vi "UHR-Fleezers Control (host) - 12.8.vi"() -> ()   [LabVIEW 2012] (continued)
                                }
                                }
                                frame #4 {
                                n2130 = Wait (ms)(milliseconds to wait=u32 500) -> ()  [unwired: 1 out]
                                }
                                frame #5 {
                                n2131 = local read "Mean"() -> (w3230:dbl)
                                n2132 = Greater?(x=w3230, y=11.0) -> (0:w3224:bool)
                                n2133 = Not(x=w3224) -> (.not. x?=w3225:bool)
                                n2134 = And(x=w3225, y="Shift confocal") -> (x .and. y?=w3227:bool)
                                n2135 = And(x=w3224, y="Shift confocal") -> (x .and. y?=w3228:bool)
                                n2136 = case shown="True" w3228 {
                                frame False {
                                }
                                frame True {
                                n2137 = local read "Confocal Y 2 (V)"() -> (w3234:dbl)
                                n2138 = local read "Confocal X 2 (V)"() -> (w3233:dbl)
                                n2139 = property on="AO1" class="Slide (strict)"("Val(Sgnl)"=w3234) -> ()  [unwired: 2 in, 2 out]
                                n2140 = property on="AO2" class="Slide (strict)"("Val(Sgnl)"=w3233) -> ()  [unwired: 2 in, 2 out]
                                }
                                }
                                n2141 = case shown="True" w3227 {
                                frame False {
                                }
                                frame True {
                                n2142 = local read "Confocal Y 1 (V)"() -> (w3232:dbl)
                                n2143 = local read "Confocal X 1 (V)"() -> (w3231:dbl)
                                n2144 = property on="AO1" class="Slide (strict)"("Val(Sgnl)"=w3232) -> ()  [unwired: 2 in, 2 out]
                                n2145 = property on="AO2" class="Slide (strict)"("Val(Sgnl)"=w3231) -> ()  [unwired: 2 in, 2 out]
                                }
                                }
                                }
                                frame #6 {
                                n2146 = Wait (ms)(milliseconds to wait=u32 1500) -> ()  [unwired: 1 out]
                                }
                                frame #7 {
                                n2147 = property on="Rem fb disp offset" class="Bool (strict)"("Val(Sgnl)"=TRUE ("Value (Signaling)")) -> ()  [unwired: 2 in, 2 out]
                                }
                                }
                                }
                                frame True {
                                n2148 = flat-sequence {
                                tunnel: w3237 -> [w3238]
                                frame #0 {
                                n2149 = property on="Trap Delta (MHz)" class="DigNum (strict)"("Val(Sgnl)"=w3238) -> ()  [unwired: 2 in, 2 out]
                                }
                                frame #1 {
                                n2150 = Wait (ms)(milliseconds to wait=u32 500) -> ()  [unwired: 1 out]
                                }
                                frame #2 {
                                n2151 = local read "Shift confocal"() -> (w3244:bool)
                                n2152 = local read "Mean"() -> (w3246:dbl)
                                n2153 = Greater?(x=w3246, y=11.0) -> (0:w3243:bool)
                                n2154 = Not(x=w3243) -> (.not. x?=w3242:bool)
                                n2155 = And(x=w3242, y=w3244) -> (x .and. y?=w3240:bool)
                                n2156 = And(x=w3243, y=w3244) -> (x .and. y?=w3241:bool)
                                n2157 = case shown="True" w3241 {
                                frame False {
                                }
                                frame True {
                                n2158 = local read "Confocal Y 2 (V)"() -> (w3250:dbl)
                                n2159 = local read "Confocal X 2 (V)"() -> (w3249:dbl)
                                n2160 = property on="AO2" class="Slide (strict)"("Val(Sgnl)"=w3249) -> ()  [unwired: 2 in, 2 out]
                                n2161 = property on="AO1" class="Slide (strict)"("Val(Sgnl)"=w3250) -> ()  [unwired: 2 in, 2 out]
                                }
                                }
                                n2162 = case shown="True" w3240 {
                                frame False {
                                }
                                frame True {
                                n2163 = local read "Confocal X 1 (V)"() -> (w3247:dbl)
                                n2164 = local read "Confocal Y 1 (V)"() -> (w3248:dbl)
                                n2165 = property on="AO2" class="Slide (strict)"("Val(Sgnl)"=w3247) -> ()  [unwired: 2 in, 2 out]
                                n2166 = property on="AO1" class="Slide (strict)"("Val(Sgnl)"=w3248) -> ()  [unwired: 2 in, 2 out]
                                }
                                }
                                }
                                }
                                }
                                }
                                }
                                }
                                }
                                frame "Image" {
                                n2167 = property on="Confocal Image" class="Bool (strict)"("Val(Sgnl)"=TRUE ("Value (Signaling)")) -> ()  [unwired: 2 in, 2 out]
                                }
                              }
                              n2168 = local write "Fl. High"(FALSE ("Fl. High")) -> ()
                              n2169 = local read "Time (s)"() -> (w3184:dbl)
                            }
                            frame #1 {
                              n2170 = case shown="True" "Auto F Reset" {
                                tunnel: w3256 -> [_ w3261]
                                tunnel: w3255 -> [_ w3260]
                                tunnel: w3254 -> [_ w3259]
                                tunnel: w3253 -> [_ w3258]
                                frame False {
                                }
                                frame True {
                                n2171 = node-c288() -> (w3263:T23)  [unwired: 4 in]
                                n2172 = timed-loop {
                                timing: w3263 -> [_]
                                timing-out: [_] -> w3262
                                tunnel: w3261 -> [w3268]
                                tunnel: w3260 -> [w3267]
                                tunnel: w3259 -> [w3266]
                                tunnel: w3258 -> [w3265]
                                stop <- w3264 stop-if-true
                                n2173 = node-c288() -> ()  [unwired: 1 in, 1 out]
                                n2174 = local read "Fl. Delta Thresh. (kHz)"() -> (w3277:dbl)
                                n2175 = local read "APD to Watch"() -> (w3278:bool)
                                n2176 = local read "Delta Fl. 1"() -> (w3279:dbl)
                                n2177 = local read "Delta Fl. 2"() -> (w3280:dbl)
                                n2178 = local read "Fl. Triggered..."() -> (w3271:bool)
                                n2179 = local read "Stop All"() -> (w3272:bool)
                                n2180 = local read "Reset Force"() -> (w3270:bool)
                                n2181 = Multiply(x=w3277, y=1000.0) -> (x*y=w3275:dbl)
                                n2182 = Select(t=w3279, s=w3278, f=w3280) -> (s? t:f=w3274:dbl)
                                n2183 = Not(x=w3271) -> (.not. x?=w3269:bool)
                                n2184 = Greater?(x=w3274, y=w3275) -> (0:w3273:bool)
                                n2185 = Compound Arithmetic op=OR(w3273, w3272, w3269, w3270) -> (w3264:bool)
                                n2186 = case shown="True" w3264 {
                                tunnel: w3268 -> [_ w3284]
                                tunnel: w3267 -> [_ w3288]
                                tunnel: w3266 -> [_ w3287]
                                tunnel: w3265 -> [_ w3286]
                                frame False {
                                }
                                frame True {
                                n2187 = case shown="\"Yank\"" w3288 {
                                tunnel: w3287 -> [_ w3298]
                                tunnel: w3286 -> [_ w3296]
                                frame "Image", Default {
                                }
                                frame "Yank" {
                                n2188 = flat-sequence {
                                tunnel: [w3301] -> w3299
                                tunnel: w3298 -> [w3301]
                                tunnel: [w3300] -> w3297
                                tunnel: w3296 -> [w3300]
                                tunnel: w3299 -> [w3307]
                                tunnel: w3297 -> [w3305]
                                frame #0 {
                                n2189 = local read "Yank Delay (s)"() -> (w3304:dbl)
                                n2190 = Multiply(x=w3304, y=1000.0) -> (x*y=w3302:dbl)
                                n2191 = Wait (ms)(milliseconds to wait=w3302) -> ()  [unwired: 1 out]
                                }
                                frame #1 {
                                n2192 = local read "Yank to which?"() -> (w3306:bool)
                                n2193 = case shown="False" w3306 {
                                tunnel: w3307 -> [_ w3335]
                                tunnel: w3305 -> [w3308 _]
                                frame False {
                                n2194 = flat-sequence {
                                tunnel: w3308 -> [w3309]
                                frame #0 {
                                n2195 = property on="Trap Pos FB SP" class="DigNum (strict)"("Val(Sgnl)"=w3309) -> ()  [unwired: 2 in, 2 out]
                                }
                                frame #1 {
                                n2196 = Wait (ms)(milliseconds to wait=u32 700) -> ()  [unwired: 1 out]
                                }
                                frame #2 {
                                n2197 = local read "Action (%)"() -> (w3314:dbl)
                                n2198 = Absolute Value(x=w3314) -> (abs(x)=w3313:dbl)
                                n2199 = Greater?(x=w3313, y=70.0) -> (0:w3311:bool)
                                n2200 = property on="Remove Action Offset" class="Bool (strict)"("Val(Sgnl)"=w3311) -> ()  [unwired: 2 in, 2 out]
                                }
                                frame #3 {
                                n2201 = for {
                                N: 4 -> [_]
                                n2202 = flat-sequence {
                                frame #0 {
                                n2203 = Wait (ms)(milliseconds to wait=u32 500) -> ()  [unwired: 1 out]
                                }
                                frame #1 {
                                n2204 = local read "Action (%)"() -> (w3320:dbl)
                                n2205 = Absolute Value(x=w3320) -> (abs(x)=w3319:dbl)
                                n2206 = Greater?(x=w3319, y=70.0) -> (0:w3317:bool)
                                n2207 = property on="Remove Action Offset" class="Bool (strict)"("Val(Sgnl)"=w3317) -> ()  [unwired: 2 in, 2 out]
                                }
                                }
                                }
                                }
                                frame #4 {
                                n2208 = Wait (ms)(milliseconds to wait=u32 500) -> ()  [unwired: 1 out]
                                }
                                frame #5 {
                                n2209 = local read "Shift confocal"() -> (w3325:bool)
                                n2210 = local read "Mean"() -> (w3328:dbl)
                                n2211 = Greater?(x=w3328, y=11.0) -> (0:w3324:bool)
                                n2212 = Not(x=w3324) -> (.not. x?=w3323:bool)
                                n2213 = And(x=w3324, y=w3325) -> (x .and. y?=w3326:bool)
                                n2214 = And(x=w3323, y=w3325) -> (x .and. y?=w3322:bool)
                                n2215 = case shown="True" w3326 {
                                frame False {
                                }
                                frame True {
                                n2216 = local read "Confocal X 2 (V)"() -> (w3331:dbl)
                                n2217 = local read "Confocal Y 2 (V)"() -> (w3332:dbl)
                                n2218 = property on="AO2" class="Slide (strict)"("Val(Sgnl)"=w3331) -> ()  [unwired: 2 in, 2 out]
                                n2219 = property on="AO1" class="Slide (strict)"("Val(Sgnl)"=w3332) -> ()  [unwired: 2 in, 2 out]
                                }
                                }
                                n2220 = case shown="True" w3322 {
                                frame False {
                                }
                                frame True {
                                n2221 = local read "Confocal Y 1 (V)"() -> (w3330:dbl)
                                n2222 = local read "Confocal X 1 (V)"() -> (w3329:dbl)
                                n2223 = property on="AO1" class="Slide (strict)"("Val(Sgnl)"=w3330) -> ()  [unwired: 2 in, 2 out]
                                n2224 = property on="AO2" class="Slide (strict)"("Val(Sgnl)"=w3329) -> ()  [unwired: 2 in, 2 out]
                                }
                                }
                                }
                                frame #6 {
                                n2225 = Wait (ms)(milliseconds to wait=u32 1500) -> ()  [unwired: 1 out]
                                }
                                frame #7 {
                                n2226 = property on="Rem fb disp offset" class="Bool (strict)"("Val(Sgnl)"=TRUE ("Value (Signaling)")) -> ()  [unwired: 2 in, 2 out]
                                }
                                }
                                }
                                frame True {
                                n2227 = flat-sequence {
                                tunnel: w3335 -> [w3336]
                                frame #0 {
                                n2228 = property on="Trap Delta (MHz)" class="DigNum (strict)"("Val(Sgnl)"=w3336) -> ()  [unwired: 2 in, 2 out]
                                }
                                frame #1 {
                                n2229 = Wait (ms)(milliseconds to wait=u32 500) -> ()  [unwired: 1 out]
                                }
                                frame #2 {
                                n2230 = local read "Shift confocal"() -> (w3342:bool)
                                n2231 = local read "Mean"() -> (w3343:dbl)
                                n2232 = Greater?(x=w3343, y=11.0) -> (0:w3341:bool)
                                n2233 = And(x=w3341, y=w3342) -> (x .and. y?=w3339:bool)
                                n2234 = Not(x=w3341) -> (.not. x?=w3340:bool)
                                n2235 = And(x=w3340, y=w3342) -> (x .and. y?=w3338:bool)
                                n2236 = case shown="True" w3339 {
                                frame False {
                                }
                                frame True {
                                n2237 = local read "Confocal Y 2 (V)"() -> (w3348:dbl)
                                n2238 = local read "Confocal X 2 (V)"() -> (w3347:dbl)
                                n2239 = property on="AO1" class="Slide (strict)"("Val(Sgnl)"=w3348) -> ()  [unwired: 2 in, 2 out]
                                n2240 = property on="AO2" class="Slide (strict)"("Val(Sgnl)"=w3347) -> ()  [unwired: 2 in, 2 out]
                                }
                                }
                                n2241 = case shown="True" w3338 {
                                frame False {
                                }
                                frame True {
                                n2242 = local read "Confocal Y 1 (V)"() -> (w3346:dbl)
                                n2243 = local read "Confocal X 1 (V)"() -> (w3345:dbl)
                                n2244 = property on="AO2" class="Slide (strict)"("Val(Sgnl)"=w3345) -> ()  [unwired: 2 in, 2 out]
                                n2245 = property on="AO1" class="Slide (strict)"("Val(Sgnl)"=w3346) -> ()  [unwired: 2 in, 2 out]
                                }
                                }
                                }
                                }
                                }
                                }
                                }
                                }
                                }
                                }
                                n2246 = local read "Time (s)"() -> (w3283:dbl)
                                n2247 = Subtract(x=w3284, y=w3283) -> (x-y=w3295:dbl)
                                n2248 = Number To Decimal String(number=w3295, width (-)=i16 0) -> (decimal integer string=w3293:string)
                                n2249 = Concatenate Strings(w3293, " s fluorescence event") -> (w3290:string)
                                n2250 = local read "Messages"() -> (w3291:string)
                                n2251 = local write "Duration (s)"(w3295) -> ()
                                n2252 = call "Update messages.vi"("Message to add"=w3290, "Old message string"=w3291) -> ("New message string"=w3289:string)
                                n2253 = local write "Messages"(w3289) -> ()
                                n2254 = call <vilib>:"Beep.vi"() -> ()  [unwired: 12 in]
                                n2255 = local write "Reset Force"(FALSE ("Force Reset")) -> ()
                                n2256 = local write "Fl. High"(TRUE ("Fl. High")) -> ()
                                n2257 = local write "Waiting"(TRUE ("Waiting")) -> ()
                                }
                                }
                                n2258 = node-c288() -> ()  [unwired: 1 in, 1 out]
                                }
                                n2259 = node-c288(w3262) -> ()  [unwired: 1 out]
                                }
                              }
                            }
                          }
                          n2260 = local read "Trap Delta (MHz)"() -> (w3174:dbl)
                          n2261 = local read "Trap Pos FB SP"() -> (w3172:fxp<+/-,16,1>)
                        }
                      }
                    }
                    frame True {
                      n2262 = flat-sequence {
                        tunnel: w3359 -> [w3369]
                        tunnel: [w3369] -> w3363
                        tunnel: w3362 -> [w3368]
                        tunnel: [w3368] -> w3361
                        tunnel: [w3367] -> w3360
                        tunnel: w3358 -> [w3366]
                        tunnel: [w3365] -> w3357
                        tunnel: w3354 -> [w3364]
                        tunnel: [w3364] -> w3353
                        tunnel: w3363 -> [w3439]
                        tunnel: w3361 -> [w3438]
                        tunnel: w3360 -> [w3437]
                        tunnel: w3357 -> [w3436]
                        tunnel: w3353 -> [w3435]
                        tunnel: [w3436] -> w3356
                        frame #0 {
                          n2263 = call <vilib>:"Beep.vi"() -> ()  [unwired: 3 in, 9 out]
                          n2264 = local write "Waiting"(FALSE ("Waiting")) -> ()
                          n2265 = Increment(x=w3366) -> (x+1=w3365:u8)
                          n2266 = case shown="\"Yank\"" w3368 {
                            tunnel: w3365 -> [_ _ w3375]
                            frame "Image" {
                              n2267 = property on="Confocal Image" class="Bool (strict)"("Val(Sgnl)"=TRUE ("Value (Signaling)")) -> ()  [unwired: 2 in, 2 out]
                            }
                            frame "Alarm", Default {
                            }
                            frame "Yank" {
                              n2268 = flat-sequence {
                                tunnel: w3375 -> [w3378]
                                tunnel: [w3377] -> w3374
                                tunnel: ["N Array El"] -> w3373
                                tunnel: w3374 -> [w3392]
                                tunnel: w3373 -> [w3388]
                                frame #0 {
                                n2269 = Multiply(x="Yank Delay (s)", y=1000.0) -> (x*y=w3381:dbl)
                                n2270 = Quotient & Remainder(x=w3378, y="N Array El") -> (x-y*floor(x/y)=w3377:u8)  [unwired: 1 out]
                                n2271 = Wait (ms)(milliseconds to wait=w3381) -> ()  [unwired: 1 out]
                                }
                                frame #1 {
                                n2272 = Random Number (0-1)() -> (number: 0 to 1=w3389:dbl)
                                n2273 = Multiply(x=w3388, y=w3389) -> (x*y=w3387:dbl)
                                n2274 = Round Toward -Infinity(1:w3387) -> (0:w3386:dbl)
                                n2275 = Select(t=w3386, s="Random Choice", f=w3392) -> (s? t:f=w3390:dbl)
                                n2276 = Select(t="Yank to Trap Delta (MHz)", s="Yank to which?", f="Yank to SP") -> (s? t:f=w3383:dbl[])
                                n2277 = Index Array(array=w3383, index=w3390) -> (element=w3393:dbl)
                                n2278 = case shown="False" "Yank to which?" {
                                tunnel: w3393 -> [w3394 w3420]
                                frame False {
                                n2279 = flat-sequence {
                                tunnel: w3394 -> [w3395]
                                frame #0 {
                                n2280 = property on="Trap Pos FB SP" class="DigNum (strict)"("Val(Sgnl)"=w3395) -> ()  [unwired: 2 in, 2 out]
                                }
                                frame #1 {
                                n2281 = Wait (ms)(milliseconds to wait=u32 700) -> ()  [unwired: 1 out]
                                }
                                frame #2 {
                                n2282 = local read "Action (%)"() -> (w3400:dbl)
                                n2283 = Absolute Value(x=w3400) -> (abs(x)=w3399:dbl)
                                n2284 = Greater?(x=w3399, y=70.0) -> (0:w3397:bool)
                                n2285 = property on="Remove Action Offset" class="Bool (strict)"("Val(Sgnl)"=w3397) -> ()  [unwired: 2 in, 2 out]
                                }
                                frame #3 {
                                n2286 = for {
                                N: 4 -> [_]
                                n2287 = flat-sequence {
                                frame #0 {
                                n2288 = Wait (ms)(milliseconds to wait=u32 500) -> ()  [unwired: 1 out]
                                }
                                frame #1 {
                                n2289 = local read "Action (%)"() -> (w3406:dbl)
                                n2290 = Absolute Value(x=w3406) -> (abs(x)=w3405:dbl)
                                n2291 = Greater?(x=w3405, y=70.0) -> (0:w3403:bool)
                                n2292 = property on="Remove Action Offset" class="Bool (strict)"("Val(Sgnl)"=w3403) -> ()  [unwired: 2 in, 2 out]
                                }
                                }
                                }
                                }
                                frame #4 {
                                n2293 = local read "Shift confocal"() -> (w3410:bool)
                                n2294 = local read "Mean"() -> (w3413:dbl)
                                n2295 = Greater?(x=w3413, y=11.0) -> (0:w3409:bool)
                                n2296 = Not(x=w3409) -> (.not. x?=w3408:bool)
                                n2297 = And(x=w3408, y=w3410) -> (x .and. y?=w3407:bool)
                                n2298 = And(x=w3409, y=w3410) -> (x .and. y?=w3411:bool)
                                n2299 = case shown="True" w3411 {
                                frame False {
                                }
                                frame True {
                                n2300 = local read "Confocal X 2 (V)"() -> (w3416:dbl)
                                n2301 = local read "Confocal Y 2 (V)"() -> (w3417:dbl)
                                n2302 = property on="AO2" class="Slide (strict)"("Val(Sgnl)"=w3416) -> ()  [unwired: 2 in, 2 out]
                                n2303 = property on="AO1" class="Slide (strict)"("Val(Sgnl)"=w3417) -> ()  [unwired: 2 in, 2 out]
                                }
                                }
                                n2304 = case shown="True" w3407 {
                                frame False {
                                }
                                frame True {
                                n2305 = local read "Confocal X 1 (V)"() -> (w3414:dbl)
                                n2306 = local read "Confocal Y 1 (V)"() -> (w3415:dbl)
                                n2307 = property on="AO1" class="Slide (strict)"("Val(Sgnl)"=w3415) -> ()  [unwired: 2 in, 2 out]
                                n2308 = property on="AO2" class="Slide (strict)"("Val(Sgnl)"=w3414) -> ()  [unwired: 2 in, 2 out]
                                }
                                }
                                }
                                frame #5 {
                                n2309 = Wait (ms)(milliseconds to wait=u32 1500) -> ()  [unwired: 1 out]
                                }
                                frame #6 {
                                n2310 = property on="Rem fb disp offset" class="Bool (strict)"("Val(Sgnl)"=TRUE ("Value (Signaling)")) -> ()  [unwired: 2 in, 2 out]
                                }
                                }
                                }
                                frame True {
                                n2311 = flat-sequence {
                                tunnel: w3420 -> [w3421]
                                frame #0 {
                                n2312 = property on="Trap Delta (MHz)" class="DigNum (strict)"("Val(Sgnl)"=w3421) -> ()  [unwired: 2 in, 2 out]
                                }
                                frame #1 {
                                n2313 = Wait (ms)(milliseconds to wait=u32 500) -> ()  [unwired: 1 out]
                                }
                                frame #2 {
                                n2314 = local read "Shift confocal"() -> (w3425:bool)
                                n2315 = local read "Mean"() -> (w3423:dbl)
                                n2316 = Greater?(x=w3423, y=11.0) -> (0:w3426:bool)
                                n2317 = Not(x=w3426) -> (.not. x?=w3427:bool)
                                n2318 = And(x=w3427, y=w3425) -> (x .and. y?=w3429:bool)
                                n2319 = And(x=w3426, y=w3425) -> (x .and. y?=w3428:bool)
                                n2320 = case shown="True" w3428 {
                                frame False {
                                }
                                frame True {
                                n2321 = local read "Confocal Y 2 (V)"() -> (w3433:dbl)
                                n2322 = local read "Confocal X 2 (V)"() -> (w3432:dbl)
                                n2323 = property on="AO1" class="Slide (strict)"("Val(Sgnl)"=w3433) -> ()  [unwired: 2 in, 2 out]
                                n2324 = property on="AO2" class="Slide (strict)"("Val(Sgnl)"=w3432) -> ()  [unwired: 2 in, 2 out]
                                }
                                }
                                n2325 = case shown="True" w3429 {
                                frame False {
                                }
                                frame True {
                                n2326 = local read "Confocal X 1 (V)"() -> (w3430:dbl)
                                n2327 = local read "Confocal Y 1 (V)"() -> (w3431:dbl)
                                n2328 = property on="AO2" class="Slide (strict)"("Val(Sgnl)"=w3430) -> ()  [unwired: 2 in, 2 out]
                                n2329 = property on="AO1" class="Slide (strict)"("Val(Sgnl)"=w3431) -> ()  [unwired: 2 in, 2 out]
                                }
                                }
                                }
                                }
                                }
                                }
                                }
                              }
                            }
                          }
                          n2330 = local read "Time (s)"() -> (w3367:dbl)
                          "Fl. High" <- TRUE ("Yanking")
                        }
                        frame #1 {
                          n2331 = local read "Auto F Reset"() -> (w3434:bool)
                          n2332 = case shown="True" w3434 {
                            tunnel: w3439 -> [_ w3443]
                            tunnel: w3438 -> [_ w3442]
                            tunnel: w3437 -> [_ w3441]
                            tunnel: w3435 -> [_ w3440]
                            frame False {
                            }
                            frame True {
                              n2333 = node-c288() -> (w3445:T23)  [unwired: 4 out]
                              n2334 = timed-loop {
                                timing: w3445 -> [_]
                                timing-out: [_] -> w3444
                                tunnel: w3443 -> [w3463]
                                tunnel: w3442 -> [w3462]
                                tunnel: w3441 -> [w3461]
                                tunnel: w3440 -> [w3460]
                                stop <- w3446 stop-if-true
                                n2335 = node-c288() -> ()  [unwired: 2 out]
                                n2336 = local read "Fl. Delta Thresh. (kHz)"() -> (w3454:dbl)
                                n2337 = local read "Fl. Triggered..."() -> (w3459:bool)
                                n2338 = local read "Delta Fl. 1"() -> (w3450:dbl)
                                n2339 = local read "Delta Fl. 2"() -> (w3448:dbl)
                                n2340 = local read "Stop All"() -> (w3457:bool)
                                n2341 = local read "APD to Watch"() -> (w3449:bool)
                                n2342 = Select(t=w3450, s=w3449, f=w3448) -> (s? t:f=w3447:dbl)
                                n2343 = Not(x=w3459) -> (.not. x?=w3458:bool)
                                n2344 = Multiply(x=w3454, y=1000.0) -> (x*y=w3453:dbl)
                                n2345 = Negate(x=w3453) -> (-x=w3452:dbl)
                                n2346 = Less?(x=w3447, y=w3452) -> (x < y?=w3456:bool)
                                n2347 = Compound Arithmetic op=OR(w3456, w3457, w3458, "Reset Force") -> (w3446:bool)
                                n2348 = case shown="True" w3446 {
                                tunnel: w3463 -> [_ w3478]
                                tunnel: w3462 -> [_ w3477]
                                tunnel: w3461 -> [_ w3467]
                                tunnel: w3460 -> [_ w3469]
                                frame False {
                                }
                                frame True {
                                n2349 = local read "Time (s)"() -> (w3468:dbl)
                                n2350 = case shown="\"Yank\"" w3477 {
                                tunnel: w3478 -> [_ w3481]
                                tunnel: w3469 -> [_ w3479]
                                frame "Image", Default {
                                }
                                frame "Yank" {
                                n2351 = flat-sequence {
                                tunnel: [w3487] -> w3482
                                tunnel: w3481 -> [w3487]
                                tunnel: [w3483] -> w3480
                                tunnel: w3479 -> [w3483]
                                tunnel: w3482 -> [w3490]
                                tunnel: w3480 -> [w3488]
                                frame #0 {
                                n2352 = local read "Yank Delay (s)"() -> (w3486:dbl)
                                n2353 = Multiply(x=w3486, y=1000.0) -> (x*y=w3484:dbl)
                                n2354 = Wait (ms)(milliseconds to wait=w3484) -> ()  [unwired: 1 out]
                                }
                                frame #1 {
                                n2355 = local read "Yank to which?"() -> (w3489:bool)
                                n2356 = case shown="False" w3489 {
                                tunnel: w3490 -> [_ w3517]
                                tunnel: w3488 -> [w3491 _]
                                frame False {
                                n2357 = flat-sequence {
                                tunnel: w3491 -> [w3492]
                                frame #0 {
                                n2358 = property on="Trap Pos FB SP" class="DigNum (strict)"("Val(Sgnl)"=w3492) -> ()  [unwired: 2 in, 2 out]
                                }
                                frame #1 {
                                n2359 = Wait (ms)(milliseconds to wait=u32 700) -> ()  [unwired: 1 out]
                                }
                                frame #2 {
                                n2360 = local read "Action (%)"() -> (w3497:dbl)
                                n2361 = Absolute Value(x=w3497) -> (abs(x)=w3496:dbl)
                                n2362 = Greater?(x=w3496, y=70.0) -> (0:w3494:bool)
                                n2363 = property on="Remove Action Offset" class="Bool (strict)"("Val(Sgnl)"=w3494) -> ()  [unwired: 2 in, 2 out]
                                }
                                frame #3 {
                                n2364 = for {
                                N: 4 -> [_]
                                n2365 = flat-sequence {
                                frame #0 {
                                n2366 = Wait (ms)(milliseconds to wait=u32 500) -> ()  [unwired: 1 out]
                                }
                                frame #1 {
                                n2367 = local read "Action (%)"() -> (w3503:dbl)
                                n2368 = Absolute Value(x=w3503) -> (abs(x)=w3502:dbl)
                                n2369 = Greater?(x=w3502, y=70.0) -> (0:w3500:bool)
                                n2370 = property on="Remove Action Offset" class="Bool (strict)"("Val(Sgnl)"=w3500) -> ()  [unwired: 2 in, 2 out]
                                }
                                }
                                }
                                }
                                frame #4 {
                                n2371 = local read "Shift confocal"() -> (w3508:bool)
                                n2372 = local read "Mean"() -> (w3510:dbl)
                                n2373 = Greater?(x=w3510, y=11.0) -> (0:w3507:bool)
                                n2374 = Not(x=w3507) -> (.not. x?=w3506:bool)
                                n2375 = And(x=w3507, y=w3508) -> (x .and. y?=w3505:bool)
                                n2376 = And(x=w3506, y=w3508) -> (x .and. y?=w3504:bool)
                                n2377 = case shown="True" w3505 {
                                frame False {
                                }
                                frame True {
                                n2378 = local read "Confocal Y 2 (V)"() -> (w3514:dbl)
                                n2379 = local read "Confocal X 2 (V)"() -> (w3513:dbl)
                                n2380 = property on="AO2" class="Slide (strict)"("Val(Sgnl)"=w3513) -> ()  [unwired: 2 in, 2 out]
                                n2381 = property on="AO1" class="Slide (strict)"("Val(Sgnl)"=w3514) -> ()  [unwired: 2 in, 2 out]
                                }
                                }
                                n2382 = case shown="True" w3504 {
                                frame False {
                                }
                                frame True {
                                n2383 = local read "Confocal X 1 (V)"() -> (w3511:dbl)
                                n2384 = local read "Confocal Y 1 (V)"() -> (w3512:dbl)
                                n2385 = property on="AO1" class="Slide (strict)"("Val(Sgnl)"=w3512) -> ()  [unwired: 2 in, 2 out]
                                n2386 = property on="AO2" class="Slide (strict)"("Val(Sgnl)"=w3511) -> ()  [unwired: 2 in, 2 out]
                                }
                                }
                                }
                                frame #5 {
                                n2387 = Wait (ms)(milliseconds to wait=u32 1500) -> ()  [unwired: 1 out]
                                }
                                frame #6 {
                                n2388 = property on="Rem fb disp offset" class="Bool (strict)"("Val(Sgnl)"=TRUE ("Value (Signaling)")) -> ()  [unwired: 2 in, 2 out]
                                }
                                }
                                }
                                frame True {
                                n2389 = flat-sequence {
                                tunnel: w3517 -> [w3518]
                                frame #0 {
                                n2390 = property on="Trap Delta (MHz)" class="DigNum (strict)"("Val(Sgnl)"=w3518) -> ()  [unwired: 2 in, 2 out]
                                }
                                frame #1 {
                                n2391 = Wait (ms)(milliseconds to wait=u32 500) -> ()  [unwired: 1 out]
                                }
                                frame #2 {
                                n2392 = local read "Shift confocal"() -> (w3524:bool)
                                n2393 = local read "Mean"() -> (w3526:dbl)
                                n2394 = Greater?(x=w3526, y=11.0) -> (0:w3523:bool)
                                n2395 = Not(x=w3523) -> (.not. x?=w3522:bool)
                                n2396 = And(x=w3523, y=w3524) -> (x .and. y?=w3521:bool)
                                n2397 = And(x=w3522, y=w3524) -> (x .and. y?=w3520:bool)
                                n2398 = case shown="True" w3521 {
                                frame False {
                                }
                                frame True {
                                n2399 = local read "Confocal Y 2 (V)"() -> (w3530:dbl)
                                n2400 = local read "Confocal X 2 (V)"() -> (w3529:dbl)
                                n2401 = property on="AO2" class="Slide (strict)"("Val(Sgnl)"=w3529) -> ()  [unwired: 2 in, 2 out]
                                n2402 = property on="AO1" class="Slide (strict)"("Val(Sgnl)"=w3530) -> ()  [unwired: 2 in, 2 out]
                                }
                                }
                                n2403 = case shown="True" w3520 {
                                frame False {
                                }
                                frame True {
                                n2404 = local read "Confocal Y 1 (V)"() -> (w3528:dbl)
                                n2405 = local read "Confocal X 1 (V)"() -> (w3527:dbl)
                                n2406 = property on="AO2" class="Slide (strict)"("Val(Sgnl)"=w3527) -> ()  [unwired: 2 in, 2 out]
                                n2407 = property on="AO1" class="Slide (strict)"("Val(Sgnl)"=w3528) -> ()  [unwired: 2 in, 2 out]
                                }
                                }
                                }
                                }
                                }
                                }
                                }
                                }
                                }
                                }
                                n2408 = local read "Messages"() -> (w3476:string)
                                n2409 = Subtract(x=w3468, y=w3467) -> (x-y=w3474:dbl)
                                "Duration (s)" <- w3474
                                n2410 = Number To Decimal String(number=w3474, width (-)=i16 0) -> (decimal integer string=w3472:string)
                                n2411 = Concatenate Strings(w3472, " s fluorescence event." ("string")) -> (w3470:string)
                                n2412 = call "Update messages.vi"("Message to add"=w3470, "Old message string"=w3476) -> ("New message string"=w3475:string)
                                n2413 = local write "Reset Force"(FALSE ("Reset Force")) -> ()
                                n2414 = local write "Waiting"(TRUE ("Waiting")) -> ()
                                n2415 = local write "Messages"(w3475) -> ()
                                n2416 = local write "Fl. High"(FALSE ("Fl. High")) -> ()
                                n2417 = call <vilib>:"Beep.vi"() -> ()  [unwired: 3 in, 9 out]
                                }
                                }
                                n2418 = node-c288() -> ()  [unwired: 2 out]
                              }
                              n2419 = node-c288(w3444) -> ()  [unwired: 1 out]
                            }
                          }
                        }
                      }
                      n2420 = local read "Trap Delta (MHz)"() -> (w3359:dbl)
                      n2421 = local read "Trap Pos FB SP"() -> (w3354:fxp<+/-,16,1>)
                    }
                  }
                }
                frame #1 {
                  n2422 = local read "Stop All"() -> (w3540:bool)
                  n2423 = local read "Fl. Triggered..."() -> (w3538:bool)
                  n2424 = Not(x=w3538) -> (.not. x?=w3539:bool)
                  n2425 = Or(x=w3539, y=w3540) -> (x .or. y?=w3537:bool)
                }
              }
              n2426 = case shown="True" w3131 {
                frame False {
                }
                frame True {
                  n2427 = local read "Confocal Y 1 (V)"() -> (w3141:dbl)
                  n2428 = local read "Confocal X 1 (V)"() -> (w3140:dbl)
                  n2429 = property on="AO2" class="Slide (strict)"("Val(Sgnl)"=w3140) -> ()  [unwired: 2 in, 2 out]
                  n2430 = property on="AO1" class="Slide (strict)"("Val(Sgnl)"=w3141) -> ()  [unwired: 2 in, 2 out]
                }
              }
              n2431 = case shown="True" w3131 {
                frame False {
                }
                frame True {
                  w3139 = FALSE ("Fl. High")
                  n2432 = local write "Waiting"(w3139) -> ()
                  n2433 = local write "Fl. High"(w3139) -> ()
                }
              }
              n2434 = node-c288() -> ()  [unwired: 2 out]
            }
            n2435 = node-c288(w3129) -> ()  [unwired: 1 out]
          }
        }
      }
      event "Stop All": Value Change {
        n2436 = event-data() -> ()  [unwired: 7 out]
        n2437 = local read "Stop All"() -> (w3545:bool)
      }
    }
    n2438 = node-c288() -> ()  [unwired: 2 out]
  }
  n2439 = node-c288(i64 1 ("Period"), 1 ("Processor")) -> (w73:T23)  [unwired: 2 out]
  n2440 = timed-loop "Main data acquisition loop (get data, process data for display, and save data to disk)" {
    tunnel: w11 -> [w3867]
    tunnel: w10 -> [w3866]
    tunnel: [w3895] -> w80
    tunnel: [w3890] -> w79
    timing: w73 -> [_]
    timing-out: [_] -> w72
    tunnel: w47 -> [w3727]
    stop <- "Stop All" stop-if-true
    w3644 = "Initialize"
    # "T2 sum"
    # "T1 sum"
    # "Fluorescence data into FIFO for external control vi's\n(e.g., fluorescence triggering) - Duncan Nall"
    n2441 = node-c288() -> ()  [unwired: 2 out]
    n2442 = First Call?() -> (First Call?: T/F=w3679:bool)
    n2443 = Or(x="Reset", y=w3679) -> (x .or. y?=w3680:bool)
    n2444 = local read "Flushing P1"() -> (w3599:bool)
    n2445 = case "Reset data stream (manual reset or at begining of some rastering and imaging)" shown="True" w3680 {
      tunnel: w3867 -> [w4959 w4967]
      tunnel: w3866 -> [w4958 w4966]
      tunnel: [w4959 w4961] -> w3862
      tunnel: [w4958 w4960] -> w3861
      frame False {
      }
      frame True {
        w4964 = TRUE ("AI to FIFO")
        n2446 = local write "Overflow (data lost)"(FALSE ("Overflow (data lost)")) -> ()
        n2447 = call "reset FPGA DMA.vi"("error in"=w4966, "FPGA VI Reference In"=w4967) -> ("error out"=w4962:errorcluster, "FPGA VI Reference Out"=w4963:T20)
        n2448 = xnode "Read/Write Control"("FPGA VI Reference In"=w4963, "error in"=w4962, "AI to FIFO"=w4964, "APD to FIFO"=w4964) -> ("FPGA VI Reference Out"=w4961:T20, "error out"=w4960:errorcluster)
      }
    }
    n2449 = case shown="True" w3599 {
      frame False {
      }
      frame True {
        n2450 = local read "Flush rate (uL/m) P1"() -> (w3939:dbl)
        n2451 = local read "HP1 Flush Time (s)"() -> (w3948:dbl)
        n2452 = local read "DMA Update Period (s)"() -> (w3942:dbl)
        n2453 = Divide(x=w3939, y=60.0) -> (x/y=w3940:dbl)
        n2454 = Divide(x=w3948, y=w3942) -> (x/y=w3937:dbl)
        n2455 = feedback #4(0) -> (w3946:i32)
        n2456 = Increment(x=w3946) -> (x+1=w3936:i32)
        n2457 = Greater?(x=w3936, y=w3937) -> (0:w3945:bool)
        n2458 = Compound Arithmetic op=MULTIPLY(w3942, w3936, w3940) -> (→"P1 Flush Volume (uL)":dbl)
        n2459 = Divide(x=w3936, y=w3937) -> (x/y=→"P1 Flushing Bar":dbl)
        n2460 = case shown="True" w3945 {
          tunnel: w3936 -> [w3949 _]
          tunnel: [w3949 0] -> w3944
          frame False {
          }
          frame True {
            w3950 = FALSE ("Flushing P1")
            n2461 = local write "Inject Pump 1"(w3950) -> ()
            n2462 = local write "Flushing P1"(w3950) -> ()
            n2463 = property on="Clear Volume P1" class="Bool (strict)"("Val(Sgnl)"=TRUE ("Value (Signaling)")) -> ()  [unwired: 2 in, 2 out]
          }
        }
        n2464 = feedback-in #4(w3944) -> ()
      }
    }
    n2465 = Or(x="Start AOD Scan", y="Trap Raster Scan") -> (x .or. y?=w3820:bool)
    n2466 = case "Start AOM raster scan" shown="True" w3820 {
      tunnel: w3862 -> [w4809 w4819]
      tunnel: w3861 -> [w4808 w4818]
      tunnel: [w4809 w4812] -> w3860
      tunnel: [w4808 w4811] -> w3859
      frame False {
      }
      frame True {
        n2467 = case shown="True" "Restart DMA? (AOD)" {
          tunnel: [w4857 w4859] -> w4813
          tunnel: [w4856 w4858] -> w4814
          tunnel: w4819 -> [w4857 w4861]
          tunnel: w4818 -> [w4856 w4860]
          frame False {
          }
          frame True {
            n2468 = local write "Overflow (data lost)"(FALSE ("Overflow (data lost)")) -> ()
            n2469 = call "reset FPGA DMA.vi"("error in"=w4860, "FPGA VI Reference In"=w4861) -> ("error out"=w4858:errorcluster, "FPGA VI Reference Out"=w4859:T20)
          }
        }
        n2470 = local write "Trap Raster Scan"(FALSE ("Trap Raster Scan")) -> ()
        n2471 = case shown="True" "Move MCL Also?" {
          tunnel: w4814 -> [w4822 w4851]
          tunnel: w4813 -> [w4823 w4852]
          tunnel: [w4821 w4855] -> w4812
          tunnel: [w4820 w4854] -> w4811
          frame False {
            w4824 = TRUE ("AI to FIFO")
            n2472 = xnode "Read/Write Control"("FPGA VI Reference In"=w4823, "error in"=w4822, "AI to FIFO"=w4824, "APD to FIFO"=w4824, "Start scan"=w4824) -> ("FPGA VI Reference Out"=w4821:T20, "error out"=w4820:errorcluster)
          }
          frame True {
            w4848 = FALSE ("1D or 2D Scan?")
            w4853 = TRUE ("AI to FIFO")
            # "Count for MCL loop"
            # "N total cycles"
            # "N steps"
            # "V_int"
            n2473 = local read "Scan Range (nm)"() -> (w4830:dbl)
            n2474 = local read "Number of F/B Scans (AOD)"() -> (w4847:u16)
            n2475 = Sign(1:w4830) -> (0:w4829:dbl)
            n2476 = Compound Arithmetic op=MULTIPLY(w4830, "MCL Step Position Ratio", "MCL/AOM Scale Tweak") -> (w4834:dbl)
            n2477 = Negate(x=w4829) -> (-x=w4826:dbl)
            n2478 = Multiply(x=w4826, y="MCL Step Increment (V_int)") -> (x*y=w4828:dbl)
            n2479 = Divide(x=w4834, y="MCL X Cal (nm/V)") -> (x/y=w4840:dbl)
            n2480 = Multiply(x=32767.0 ("y"), y=w4840) -> (x*y=w4846:dbl)
            n2481 = local read "Total Counts (ticks)"() -> (w4831:u16)
            n2482 = local read "Cycles/step (AOD)"() -> (w4842:u64)
            n2483 = local read "Scan steps (AOD)"() -> (w4843:u64)
            n2484 = Divide(x=w4846, y=10.0) -> (x/y=w4839:dbl)
            n2485 = Divide(x=w4839, y="MCL Step Increment (V_int)") -> (x/y=w4837:dbl)
            n2486 = Absolute Value(x=w4837) -> (abs(x)=w4825:dbl)
            n2487 = Compound Arithmetic op=MULTIPLY(w4843, w4842, w4831) -> (w4838:u64)
            n2488 = local write "wait to reset values"(w4853) -> ()
            n2489 = local write "MCL Scanning"(w4853) -> ()
            n2490 = Divide(x=w4838, y=w4825) -> (x/y=w4835:dbl)
            "MCL Count" <- w4835
            n2491 = xnode "Read/Write Control"("FPGA VI Reference In"=w4852, "error in"=w4851, "Scan steps (MCL)"=w4825, "Number of scans (MCL)"=w4847, "Cycles per step (MCL)"=u64 1, "Scan freq.  increment (MCL)"=w4828, "1D or 2D Scan?"=w4848, "MCL Scan Axis"=w4848, "Cont. Scan (MCL)"=w4848, "MCL count"=w4835) -> ("FPGA VI Reference Out"=w4850:T20, "error out"=w4849:errorcluster)
            n2492 = xnode "Read/Write Control"("FPGA VI Reference In"=w4850, "error in"=w4849, "AI to FIFO"=w4853, "APD to FIFO"=w4853, "Start scan"=w4853, "Start scan (MCL)"=w4853) -> ("FPGA VI Reference Out"=w4855:T20, "error out"=w4854:errorcluster)
          }
        }
        "Raster Scanning..." <- TRUE ("Scanning...")
      }
    }
    n2493 = local read "Flushing P3"() -> (w3600:bool)
    n2494 = case "Keep track of when Harvard Pump 3 is done flushing" shown="True" w3600 {
      frame False {
      }
      frame True {
        n2495 = local read "Flush rate (uL/m) P3"() -> (w3956:dbl)
        n2496 = local read "DMA Update Period (s)"() -> (w3958:dbl)
        n2497 = local read "HP3 Flush Time (s)"() -> (w3965:dbl)
        n2498 = Divide(x=w3956, y=60.0) -> (x/y=w3954:dbl)
        n2499 = feedback #5(0) -> (w3963:i32)
        n2500 = Increment(x=w3963) -> (x+1=w3957:i32)
        n2501 = Divide(x=w3965, y=w3958) -> (x/y=w3959:dbl)
        n2502 = Greater?(x=w3957, y=w3959) -> (0:w3962:bool)
        n2503 = Compound Arithmetic op=MULTIPLY(w3958, w3957, w3954) -> (→"P3 Flush Volume (uL)":dbl)
        n2504 = case shown="True" w3962 {
          tunnel: w3957 -> [w3966 _]
          tunnel: [w3966 0] -> w3961
          frame False {
          }
          frame True {
            w3967 = FALSE ("Flushing P3")
            n2505 = local write "Inject Pump 3"(w3967) -> ()
            n2506 = local write "Flushing P3"(w3967) -> ()
            n2507 = property on="Clear Volume P3" class="Bool (strict)"("Val(Sgnl)"=TRUE ("Value (Signaling)")) -> ()  [unwired: 2 in, 2 out]
          }
        }
        n2508 = feedback-in #5(w3961) -> ()
        n2509 = Divide(x=w3957, y=w3959) -> (x/y=→"P3 Flushing Bar":dbl)
      }
    }
    n2510 = And(x="Save scans", y=w3820) -> (x .and. y?=w3858:bool)
    n2511 = Compound Arithmetic op=OR("Start MCL Scan", "Confocal Image", "Confocal Linescan") -> (w3818:bool)
    n2512 = And(x="Save Data (MCL)", y=w3818) -> (x .and. y?=w3857:bool)
    n2513 = case "Start MCL raster scan" shown="True" w3818 {
      tunnel: w3860 -> [w4421 w4437]
      tunnel: w3859 -> [w4420 w4436]
      tunnel: [w4421 w4432] -> w3726
      tunnel: [w4420 w4431] -> w3725
      tunnel: [FALSE w4430] -> w3843
      tunnel: "Start MCL Scan" -> [_ w4425]
      tunnel: "Confocal Image" -> [_ w4424]
      tunnel: "Confocal Linescan" -> [_ _]
      frame False {
      }
      frame True {
        w4430 = TRUE
        n2514 = case shown="True" "Restart DMA? (MCL)" {
          tunnel: [w4482 w4484] -> w4435
          tunnel: [w4481 w4483] -> w4434
          tunnel: w4437 -> [w4482 w4487]
          tunnel: w4436 -> [w4481 w4486]
          frame False {
          }
          frame True {
            n2515 = call "reset FPGA DMA.vi"("error in"=w4486, "FPGA VI Reference In"=w4487) -> ("error out"=w4483:errorcluster, "FPGA VI Reference Out"=w4484:T20)
            n2516 = local write "Overflow (data lost)"(FALSE ("Overflow (data lost)")) -> ()
          }
        }
        n2517 = case shown="False" w4425 {
          selector: w4425 -> [_ w4441]
          tunnel: w4424 -> [w4440 _]
          tunnel: [w4440 w4441] -> w4423
          frame False {
            n2518 = property on="2D or 1D Scan" class="Bool (strict)"("Val(Sgnl)"=w4440) -> ()  [unwired: 2 in, 2 out]
            n2519 = property on="Confocal Image" class="Bool (strict)"("Value"=FALSE ("Start Confocal Map")) -> ()  [unwired: 2 in, 2 out]
          }
          frame True {
          }
        }
        n2520 = local write "MCL Scanning"(w4430) -> ()
        n2521 = local read "AO1"() -> (w4427:dbl)
        n2522 = local read "AO2"() -> (w4426:dbl)
        n2523 = case shown="True" "Center Scan" {
          tunnel: w4435 -> [w4448 w4480]
          tunnel: w4434 -> [w4447 w4479]
          tunnel: [w4446 w4478] -> w4432
          tunnel: [w4445 w4477] -> w4431